vi "Dresden R2R Sputter 03.02.2018 IY24.vi"() -> ()   [LabVIEW 2009] (continued)
                                }
                                frame #1 {
                                n31817 = while {
                                i -> [w36487]
                                stop <- w36484 stop-if-true
                                n31818 = Greater?(x=w36487, y=50 ("Baratron set zero time 2")) -> (0:w36486:bool)
                                n31819 = case shown="True" w36486 {
                                frame #0 {
                                }
                                frame #1 {
                                n31820 = local write "Semi"(TRUE ("Semi")) -> ()
                                n31821 = local write "Error Message"("" ("Error Message")) -> ()
                                }
                                }
                                n31822 = local read "Pressure_ch3"() -> (w36483:i32)
                                n31823 = Less?(x=w36483, y=0.1 ("Pressure Check for baratron set zero")) -> (x < y?=w36490:bool)
                                n31824 = case shown="False" w36490 {
                                tunnel: [FALSE TRUE] -> w36489
                                frame #0 {
                                n31825 = Wait Until Next ms Multiple(millisecond multiple=u32 200) -> ()  [unwired: 1 out]
                                }
                                frame #1 {
                                }
                                }
                                n31826 = local read "Semi"() -> (w36488:bool)
                                n31827 = Or(x=w36489, y=w36488) -> (x .or. y?=w36484:bool)
                                }
                                }
                                frame #2 {
                                n31828 = local read "Semi"() -> (w36497:bool)
                                n31829 = case shown="False" w36497 {
                                frame #0 {
                                n31830 = local write "SDC1 2b"(TRUE ("SDC1 2b")) -> ()
                                n31831 = Wait (ms)(milliseconds to wait=u32 1000) -> ()  [unwired: 1 out]
                                }
                                frame #1 {
                                }
                                }
                                }
                                }
                                }
                                frame #3 {
                                # "CC CLOSE"
                                n31832 = stacked-sequence {
                                frame #0 {
                                n31833 = local read "Semi"() -> (w36500:bool)
                                n31834 = case shown="False" w36500 {
                                frame #0 {
                                n31835 = while {
                                i -> [w36506]
                                stop <- w36501 stop-if-true
                                n31836 = Greater?(x=w36506, y=50) -> (0:w36505:bool)
                                n31837 = case shown="True" w36505 {
                                frame #0 {
                                }
                                frame #1 {
                                n31838 = local write "Semi"(TRUE ("Semi")) -> ()
                                n31839 = local write "Error Message"("Coating Process  \nwas cancelled.\nPlease check \nBG-BV connection." ("Error Message")) -> ()
                                }
                                }
                                n31840 = local read "Ch3_Cc_on_off_di"() -> (w36504:bool)
                                n31841 = case shown="True" w36504 {
                                tunnel: [TRUE FALSE] -> w36503
                                frame #0 {
                                }
                                frame #1 {
                                n31842 = local write "Ch3_Cc_on_off_do"(FALSE ("Ch1_WFC_do")) -> ()
                                n31843 = Wait Until Next ms Multiple(millisecond multiple=u32 200) -> ()  [unwired: 1 out]
                                }
                                }
                                n31844 = local read "Semi"() -> (w36502:bool)
                                n31845 = Or(x=w36503, y=w36502) -> (x .or. y?=w36501:bool)
                                }
                                }
                                frame #1 {
                                }
                                }
                                }
                                frame #1 {
                                n31846 = local read "Semi"() -> (w36514:bool)
                                n31847 = case shown="False" w36514 {
                                frame #0 {
                                n31848 = local write "SDC1 3"(TRUE ("SDC1 3")) -> ()
                                n31849 = Wait (ms)(milliseconds to wait=u32 1000) -> ()  [unwired: 1 out]
                                }
                                frame #1 {
                                }
                                }
                                }
                                }
                                }
                                frame #4 {
                                # "PC-BV CLOSE"
                                n31850 = stacked-sequence {
                                frame #0 {
                                n31851 = local read "Semi"() -> (w36517:bool)
                                n31852 = case shown="False" w36517 {
                                frame #0 {
                                n31853 = stacked-sequence {
                                frame #0 {
                                n31854 = local read "Semi"() -> (w36518:bool)
                                n31855 = case shown="False" w36518 {
                                frame #0 {
                                n31856 = local write "Pc_bv3_auto_close"(TRUE ("Tp1_auto_start")) -> ()
                                }
                                frame #1 {
                                }
                                }
                                }
                                frame #1 {
                                n31857 = local read "Semi"() -> (w36520:bool)
                                n31858 = case shown="False" w36520 {
                                frame #0 {
                                n31859 = Wait (ms)(milliseconds to wait=u32 1000) -> ()  [unwired: 1 out]
                                }
                                frame #1 {
                                }
                                }
                                }
                                frame #2 {
                                n31860 = local read "Semi"() -> (w36522:bool)
                                n31861 = case shown="False" w36522 {
                                frame #0 {
                                n31862 = while {
                                i -> [w36528]
                                stop <- w36524 stop-if-true
                                n31863 = local read "Pc_bv_closed_ch3"() -> (w36526:bool)
                                n31864 = Greater?(x=w36528, y=120) -> (0:w36527:bool)
                                n31865 = local read "Semi"() -> (w36525:bool)
                                n31866 = Compound Arithmetic op=OR(w36525, w36526, w36527) -> (w36524:bool)
                                n31867 = Wait (ms)(milliseconds to wait=u32 500) -> ()  [unwired: 1 out]
                                }
                                }
                                frame #1 {
                                }
                                }
                                }
                                frame #3 {
                                n31868 = local read "Semi"() -> (w36530:bool)
                                n31869 = case shown="False" w36530 {
                                frame #0 {
                                n31870 = local read "Pc_bv_closed_ch3"() -> (w36531:bool)
                                n31871 = case shown="False" w36531 {
                                frame #0 {
                                n31872 = local write "Pc_bv3_auto_close"(TRUE ("Pc_bv1_auto_open")) -> ()
                                }
                                frame #1 {
                                }
                                }
                                }
                                frame #1 {
                                }
                                }
                                }
                                frame #4 {
                                n31873 = local read "Semi"() -> (w36533:bool)
                                n31874 = case shown="False" w36533 {
                                frame #0 {
                                n31875 = local read "Pc_bv_closed_ch3"() -> (w36534:bool)
                                n31876 = case shown="False" w36534 {
                                frame #0 {
                                n31877 = Wait (ms)(milliseconds to wait=u32 1000) -> ()  [unwired: 1 out]
                                }
                                frame #1 {
                                }
                                }
                                }
                                frame #1 {
                                }
                                }
                                }
                                frame #5 {
                                n31878 = local read "Semi"() -> (w36536:bool)
                                n31879 = case shown="False" w36536 {
                                frame #0 {
                                n31880 = while {
                                i -> [w36542]
                                stop <- w36538 stop-if-true
                                n31881 = local read "Pc_bv_closed_ch3"() -> (w36540:bool)
                                n31882 = Greater?(x=w36542, y=120) -> (0:w36541:bool)
                                n31883 = local read "Semi"() -> (w36539:bool)
                                n31884 = Compound Arithmetic op=OR(w36539, w36540, w36541) -> (w36538:bool)
                                n31885 = Wait (ms)(milliseconds to wait=u32 500) -> ()  [unwired: 1 out]
                                }
                                }
                                frame #1 {
                                }
                                }
                                }
                                frame #6 {
                                n31886 = local read "Semi"() -> (w36544:bool)
                                n31887 = case shown="False" w36544 {
                                frame #0 {
                                n31888 = local read "Pc_bv_closed_ch3"() -> (w36545:bool)
                                n31889 = case shown="False" w36545 {
                                frame #0 {
                                n31890 = local write "Error Message"("Start up process  cancelled\nbecause  PC-BV not closed.\nPlease check PC-BV1 connections." ("Error Message")) -> ()
                                n31891 = Wait (ms)(milliseconds to wait=u32 1000) -> ()  [unwired: 1 out]
                                }
                                frame #1 {
                                }
                                }
                                }
                                frame #1 {
                                }
                                }
                                }
                                }
                                }
                                frame #1 {
                                }
                                }
                                }
                                frame #1 {
                                n31892 = local read "Semi"() -> (w36548:bool)
                                n31893 = case shown="False" w36548 {
                                frame #0 {
                                n31894 = local write "SDC1 5"(TRUE ("SDC1 5")) -> ()
                                n31895 = Wait (ms)(milliseconds to wait=u32 1000) -> ()  [unwired: 1 out]
                                }
                                frame #1 {
                                }
                                }
                                }
                                }
                                }
                                frame #5 {
                                # "SOV-AR OPEN"
                                n31896 = stacked-sequence {
                                frame #0 {
                                n31897 = local read "Semi"() -> (w36551:bool)
                                n31898 = case shown="False" w36551 {
                                frame #0 {
                                n31899 = while {
                                i -> [w36557]
                                stop <- w36552 stop-if-true
                                n31900 = Greater?(x=w36557, y=50) -> (0:w36556:bool)
                                n31901 = case shown="True" w36556 {
                                frame #0 {
                                }
                                frame #1 {
                                n31902 = local write "Semi"(TRUE ("Semi")) -> ()
                                n31903 = local write "Error Message"("Coating Process  \nwas cancelled.\nPlease check \nSOV-Ar connection." ("Error Message")) -> ()
                                }
                                }
                                n31904 = local read "Ch3_Sov_Ar_di"() -> (w36555:bool)
                                n31905 = case shown="False" w36555 {
                                tunnel: [FALSE TRUE] -> w36554
                                frame #0 {
                                n31906 = local write "Ch3_Sov_Ar_do"(TRUE ("Ch1_WFC_do")) -> ()
                                n31907 = Wait Until Next ms Multiple(millisecond multiple=u32 200) -> ()  [unwired: 1 out]
                                }
                                frame #1 {
                                }
                                }
                                n31908 = local read "Semi"() -> (w36553:bool)
                                n31909 = Or(x=w36554, y=w36553) -> (x .or. y?=w36552:bool)
                                }
                                }
                                frame #1 {
                                }
                                }
                                }
                                frame #1 {
                                n31910 = local read "Semi"() -> (w36565:bool)
                                n31911 = case shown="False" w36565 {
                                frame #0 {
                                n31912 = while {
                                i -> [w36570]
                                stop <- w36568 stop-if-true
                                n31913 = Greater?(x=w36570, y=5) -> (0:w36566:bool)
                                n31914 = Wait Until Next ms Multiple(millisecond multiple=u32 1000) -> ()  [unwired: 1 out]
                                n31915 = local read "Semi"() -> (w36569:bool)
                                n31916 = Or(x=w36566, y=w36569) -> (x .or. y?=w36568:bool)
                                }
                                }
                                frame #1 {
                                }
                                }
                                }
                                frame #2 {
                                n31917 = local read "Semi"() -> (w36572:bool)
                                n31918 = case shown="False" w36572 {
                                frame #0 {
                                n31919 = local write "SDC1 6"(TRUE ("SDC1 6")) -> ()
                                n31920 = Wait (ms)(milliseconds to wait=u32 1000) -> ()  [unwired: 1 out]
                                }
                                frame #1 {
                                }
                                }
                                }
                                }
                                }
                                frame #6 {
                                # "CHECK CHAMBER PRESSURE"
                                n31921 = stacked-sequence {
                                frame #0 {
                                n31922 = local read "Semi"() -> (w36575:bool)
                                n31923 = case shown="False" w36575 {
                                frame #0 {
                                n31924 = while {
                                i -> [w36583]
                                stop <- w36577 stop-if-true
                                n31925 = Greater?(x=w36583, y=300) -> (0:w36582:bool)
                                n31926 = case shown="True" w36582 {
                                frame #0 {
                                }
                                frame #1 {
                                n31927 = local write "Semi"(TRUE ("Semi")) -> ()
                                n31928 = local write "Error Message"("Coating Process cancelled.\nPlease check chamber \nconnections." ("Error Message")) -> ()
                                }
                                }
                                n31929 = local read "Ch_pg_press_ch3_gui"() -> (w36576:dbl)
                                n31930 = Greater Or Equal?(x=w36576, y=0.9 ("CHAMBER PRESSURE 4")) -> (x >= y?=w36580:bool)
                                n31931 = case shown="True" w36580 {
                                tunnel: [TRUE FALSE] -> w36579
                                frame #0 {
                                }
                                frame #1 {
                                n31932 = Wait Until Next ms Multiple(millisecond multiple=u32 200) -> ()  [unwired: 1 out]
                                }
                                }
                                n31933 = local read "Semi"() -> (w36578:bool)
                                n31934 = Or(x=w36579, y=w36578) -> (x .or. y?=w36577:bool)
                                }
                                }
                                frame #1 {
                                }
                                }
                                }
                                frame #1 {
                                n31935 = local read "Semi"() -> (w36590:bool)
                                n31936 = case shown="False" w36590 {
                                frame #0 {
                                n31937 = Wait (ms)(milliseconds to wait=u32 1000) -> ()  [unwired: 1 out]
                                n31938 = local write "SDC1 8"(TRUE ("SDC1 8")) -> ()
                                }
                                frame #1 {
                                }
                                }
                                }
                                }
                                }
                                frame #7 {
                                # "PC-BV OPEN"
                                n31939 = stacked-sequence {
                                frame #0 {
                                n31940 = local read "Semi"() -> (w36593:bool)
                                n31941 = case shown="False" w36593 {
                                frame #0 {
                                n31942 = stacked-sequence {
                                frame #0 {
                                n31943 = local read "Semi"() -> (w36594:bool)
                                n31944 = case shown="False" w36594 {
                                frame #0 {
                                n31945 = local write "Pc_bv3_auto_open"(TRUE ("Tp1_auto_start")) -> ()
                                }
                                frame #1 {
                                }
                                }
                                }
                                frame #1 {
                                n31946 = local read "Semi"() -> (w36596:bool)
                                n31947 = case shown="False" w36596 {
                                frame #0 {
                                n31948 = Wait (ms)(milliseconds to wait=u32 1000) -> ()  [unwired: 1 out]
                                }
                                frame #1 {
                                }
                                }
                                }
                                frame #2 {
                                n31949 = local read "Semi"() -> (w36598:bool)
                                n31950 = case shown="False" w36598 {
                                frame #0 {
                                n31951 = while {
                                i -> [w36604]
                                stop <- w36600 stop-if-true
                                n31952 = local read "Pc_bv_opened_ch3"() -> (w36602:bool)
                                n31953 = Greater?(x=w36604, y=120) -> (0:w36603:bool)
                                n31954 = local read "Semi"() -> (w36601:bool)
                                n31955 = Compound Arithmetic op=OR(w36601, w36602, w36603) -> (w36600:bool)
                                n31956 = Wait (ms)(milliseconds to wait=u32 500) -> ()  [unwired: 1 out]
                                }
                                }
                                frame #1 {
                                }
                                }
                                }
                                frame #3 {
                                n31957 = local read "Semi"() -> (w36606:bool)
                                n31958 = case shown="False" w36606 {
                                frame #0 {
                                n31959 = local read "Pc_bv_opened_ch3"() -> (w36607:bool)
                                n31960 = case shown="False" w36607 {
                                frame #0 {
                                n31961 = local write "Pc_bv3_auto_open"(TRUE ("Pc_bv1_auto_open")) -> ()
                                }
                                frame #1 {
                                }
                                }
                                }
                                frame #1 {
                                }
                                }
                                }
                                frame #4 {
                                n31962 = local read "Semi"() -> (w36609:bool)
                                n31963 = case shown="False" w36609 {
                                frame #0 {
                                n31964 = local read "Pc_bv_opened_ch3"() -> (w36610:bool)
                                n31965 = case shown="False" w36610 {
                                frame #0 {
                                n31966 = Wait (ms)(milliseconds to wait=u32 1000) -> ()  [unwired: 1 out]
                                }
                                frame #1 {
                                }
                                }
                                }
                                frame #1 {
                                }
                                }
                                }
                                frame #5 {
                                n31967 = local read "Semi"() -> (w36612:bool)
                                n31968 = case shown="False" w36612 {
                                frame #0 {
                                n31969 = while {
                                i -> [w36618]
                                stop <- w36614 stop-if-true
                                n31970 = local read "Pc_bv_opened_ch3"() -> (w36616:bool)
                                n31971 = Greater?(x=w36618, y=120) -> (0:w36617:bool)
                                n31972 = local read "Semi"() -> (w36615:bool)
                                n31973 = Compound Arithmetic op=OR(w36615, w36616, w36617) -> (w36614:bool)
                                n31974 = Wait (ms)(milliseconds to wait=u32 500) -> ()  [unwired: 1 out]
                                }
                                }
                                frame #1 {
                                }
                                }
                                }
                                frame #6 {
                                n31975 = local read "Semi"() -> (w36620:bool)
                                n31976 = case shown="False" w36620 {
                                frame #0 {
                                n31977 = local read "Pc_bv_opened_ch3"() -> (w36621:bool)
                                n31978 = case shown="False" w36621 {
                                frame #0 {
                                n31979 = local write "Error Message"("Start up process  cancelled\nbecause  PC-BV not opened.\nPlease check PC-BV1 connections." ("Error Message")) -> ()
                                n31980 = Wait (ms)(milliseconds to wait=u32 1000) -> ()  [unwired: 1 out]
                                }
                                frame #1 {
                                }
                                }
                                }
                                frame #1 {
                                }
                                }
                                }
                                }
                                }
                                frame #1 {
                                }
                                }
                                }
                                frame #1 {
                                n31981 = local read "Semi"() -> (w36624:bool)
                                n31982 = case shown="False" w36624 {
                                frame #0 {
                                n31983 = Wait (ms)(milliseconds to wait=u32 1000) -> ()  [unwired: 1 out]
                                n31984 = local write "SDC1 7"(TRUE ("SDC1 7")) -> ()
                                }
                                frame #1 {
                                }
                                }
                                }
                                }
                                }
                                frame #8 {
                                # "CC OPEN"
                                n31985 = stacked-sequence {
                                frame #0 {
                                n31986 = local read "Semi"() -> (w36627:bool)
                                n31987 = case shown="False" w36627 {
                                frame #0 {
                                n31988 = while {
                                i -> [w36633]
                                stop <- w36628 stop-if-true
                                n31989 = Greater?(x=w36633, y=50) -> (0:w36632:bool)
                                n31990 = case shown="True" w36632 {
                                frame #0 {
                                }
                                frame #1 {
                                n31991 = local write "Semi"(TRUE ("Semi")) -> ()
                                n31992 = local write "Error Message"("Coating Process  \nwas cancelled.\nPlease check \nBG-BV connection." ("Error Message")) -> ()
                                }
                                }
                                n31993 = local read "Ch3_Cc_on_off_di"() -> (w36631:bool)
                                n31994 = case shown="False" w36631 {
                                tunnel: [FALSE TRUE] -> w36630
                                frame #0 {
                                n31995 = local write "Ch3_Cc_on_off_do"(TRUE ("Ch1_WFC_do")) -> ()
                                n31996 = Wait Until Next ms Multiple(millisecond multiple=u32 200) -> ()  [unwired: 1 out]
                                }
                                frame #1 {
                                }
                                }
                                n31997 = local read "Semi"() -> (w36629:bool)
                                n31998 = Or(x=w36630, y=w36629) -> (x .or. y?=w36628:bool)
                                }
                                }
                                frame #1 {
                                }
                                }
                                }
                                frame #1 {
                                n31999 = local read "Semi"() -> (w36641:bool)
                                n32000 = case shown="False" w36641 {
                                frame #0 {
                                n32001 = while {
                                i -> [w36646]
                                stop <- w36644 stop-if-true
                                n32002 = Greater?(x=w36646, y=30) -> (0:w36642:bool)
                                n32003 = Wait Until Next ms Multiple(millisecond multiple=u32 1000) -> ()  [unwired: 1 out]
                                n32004 = local read "Semi"() -> (w36645:bool)
                                n32005 = Or(x=w36642, y=w36645) -> (x .or. y?=w36644:bool)
                                }
                                }
                                frame #1 {
                                }
                                }
                                }
                                frame #2 {
                                n32006 = local read "Semi"() -> (w36648:bool)
                                n32007 = case shown="False" w36648 {
                                frame #0 {
                                n32008 = Wait (ms)(milliseconds to wait=u32 1000) -> ()  [unwired: 1 out]
                                n32009 = local write "SDC1 7b"(TRUE ("SDC1 3")) -> ()
                                }
                                frame #1 {
                                }
                                }
                                }
                                }
                                }
                                frame #9 {
                                # "CHECK CHAMBER PRESSURE"
                                n32010 = stacked-sequence {
                                frame #0 {
                                n32011 = local read "Semi"() -> (w36651:bool)
                                n32012 = case shown="False" w36651 {
                                frame #0 {
                                n32013 = while {
                                i -> [w36659]
                                stop <- w36653 stop-if-true
                                n32014 = Greater?(x=w36659, y=300) -> (0:w36658:bool)
                                n32015 = case shown="True" w36658 {
                                frame #0 {
                                }
                                frame #1 {
                                n32016 = local write "Semi"(TRUE ("Semi")) -> ()
                                n32017 = local write "Error Message"("Coating Process cancelled.\nPlease check chamber \nconnections." ("Error Message")) -> ()
                                }
                                }
                                n32018 = local read "Ch_CC_press_ch3 2"() -> (w36652:dbl)
                                n32019 = Greater Or Equal?(x=w36652, y=5e-05 ("CHAMBER PRESSURE 5")) -> (x >= y?=w36656:bool)
                                n32020 = case shown="True" w36656 {
                                tunnel: [TRUE FALSE] -> w36655
                                frame #0 {
                                }
                                frame #1 {
                                n32021 = Wait Until Next ms Multiple(millisecond multiple=u32 200) -> ()  [unwired: 1 out]
                                }
                                }
                                n32022 = local read "Semi"() -> (w36654:bool)
                                n32023 = Or(x=w36655, y=w36654) -> (x .or. y?=w36653:bool)
                                }
                                }
                                frame #1 {
                                }
                                }
                                }
                                frame #1 {
                                n32024 = local read "Semi"() -> (w36666:bool)
                                n32025 = case shown="False" w36666 {
                                frame #0 {
                                n32026 = Wait (ms)(milliseconds to wait=u32 1000) -> ()  [unwired: 1 out]
                                n32027 = local write "SDC1 10"(TRUE ("SDC1 10")) -> ()
                                }
                                frame #1 {
                                }
                                }
                                }
                                }
                                }
                                frame #10 {
                                # "CC CLOSE"
                                n32028 = stacked-sequence {
                                frame #0 {
                                n32029 = local read "Semi"() -> (w36669:bool)
                                n32030 = case shown="False" w36669 {
                                frame #0 {
                                n32031 = while {
                                i -> [w36675]
                                stop <- w36670 stop-if-true
                                n32032 = Greater?(x=w36675, y=50) -> (0:w36674:bool)
                                n32033 = case shown="True" w36674 {
                                frame #0 {
                                }
                                frame #1 {
                                n32034 = local write "Semi"(TRUE ("Semi")) -> ()
                                n32035 = local write "Error Message"("Coating Process  \nwas cancelled.\nPlease check \nBG-BV connection." ("Error Message")) -> ()
                                }
                                }
                                n32036 = local read "Ch3_Cc_on_off_di"() -> (w36673:bool)
                                n32037 = case shown="True" w36673 {
                                tunnel: [TRUE FALSE] -> w36672
                                frame #0 {
                                }
                                frame #1 {
                                n32038 = local write "Ch3_Cc_on_off_do"(FALSE ("Ch1_WFC_do")) -> ()
                                n32039 = Wait Until Next ms Multiple(millisecond multiple=u32 200) -> ()  [unwired: 1 out]
                                }
                                }
                                n32040 = local read "Semi"() -> (w36671:bool)
                                n32041 = Or(x=w36672, y=w36671) -> (x .or. y?=w36670:bool)
                                }
                                }
                                frame #1 {
                                }
                                }
                                }
                                frame #1 {
                                n32042 = local read "Semi"() -> (w36683:bool)
                                n32043 = case shown="False" w36683 {
                                frame #0 {
                                n32044 = local write "SDC1 10b"(TRUE ("SDC1 3")) -> ()
                                n32045 = Wait (ms)(milliseconds to wait=u32 1000) -> ()  [unwired: 1 out]
                                }
                                frame #1 {
                                }
                                }
                                }
                                }
                                }
                                frame #11 {
                                # "DC -Ignite Plasma"
                                n32046 = stacked-sequence {
                                frame #0 {
                                n32047 = local read "Semi"() -> (w36686:bool)
                                n32048 = case shown="False" w36686 {
                                frame #0 {
                                n32049 = stacked-sequence {
                                frame #0 {
                                n32050 = local read "Semi"() -> (w36687:bool)
                                n32051 = case shown="False" w36687 {
                                frame #0 {
                                n32052 = while {
                                i -> [w36693]
                                stop <- w36688 stop-if-true
                                n32053 = Greater?(x=w36693, y=50) -> (0:w36692:bool)
                                n32054 = case shown="True" w36692 {
                                frame #0 {
                                }
                                frame #1 {
                                n32055 = local write "Semi"(TRUE ("Semi")) -> ()
                                n32056 = local write "Error Message"("Sputtering Process cancelled.\nPlease check \nDC switch connections." ("Error Message")) -> ()
                                }
                                }
                                n32057 = local read "Cnt_Dcps_sw2_di"() -> (w36691:bool)
                                n32058 = case shown="False" w36691 {
                                tunnel: [FALSE ("Cnt_Dcps_sw1_do") TRUE ("Cnt_Dcps_sw1_do")] -> w36690
                                frame #0 {
                                n32059 = local write "Cnt_Dcps_sw2_do"(TRUE ("Cnt_Dcps_sw1_do")) -> ()
                                n32060 = Wait Until Next ms Multiple(millisecond multiple=u32 200) -> ()  [unwired: 1 out]
                                }
                                frame #1 {
                                }
                                }
                                n32061 = local read "Semi"() -> (w36689:bool)
                                n32062 = Or(x=w36690, y=w36689) -> (x .or. y?=w36688:bool)
                                }
                                }
                                frame #1 {
                                }
                                }
                                }
                                frame #1 {
                                n32063 = local read "Semi"() -> (w36701:bool)
                                n32064 = case shown="False" w36701 {
                                frame #0 {
                                n32065 = while {
                                i -> [w36707]
                                stop <- w36702 stop-if-true
                                n32066 = Greater?(x=w36707, y=50) -> (0:w36706:bool)
                                n32067 = case shown="True" w36706 {
                                frame #0 {
                                }
                                frame #1 {
                                n32068 = local write "Semi"(TRUE ("Semi")) -> ()
                                n32069 = local write "Error Message"("Sputtering Process cancelled.\nPlease check \nDC switch connections." ("Error Message")) -> ()
                                }
                                }
                                n32070 = local read "Cnt_Dcps_sw1_di"() -> (w36705:bool)
                                n32071 = case shown="True" w36705 {
                                tunnel: [TRUE ("Cnt_Dcps_sw1_do") FALSE ("Cnt_Dcps_sw1_do")] -> w36704
                                frame #0 {
                                }
                                frame #1 {
                                n32072 = local write "Cnt_Dcps_sw1_do"(FALSE ("Cnt_Dcps_sw1_do")) -> ()
                                n32073 = Wait Until Next ms Multiple(millisecond multiple=u32 200) -> ()  [unwired: 1 out]
                                }
                                }
                                n32074 = local read "Semi"() -> (w36703:bool)
                                n32075 = Or(x=w36704, y=w36703) -> (x .or. y?=w36702:bool)
                                }
                                }
                                frame #1 {
                                }
                                }
                                }
                                frame #2 {
                                n32076 = local read "Semi"() -> (w36715:bool)
                                n32077 = case shown="False" w36715 {
                                frame #0 {
                                n32078 = local write "Dc_host_auto"(TRUE ("Dc_host_auto")) -> ()
                                }
                                frame #1 {
                                }
                                }
                                }
                                frame #3 {
                                n32079 = local read "Semi"() -> (w36717:bool)
                                n32080 = case shown="False" w36717 {
                                frame #0 {
                                n32081 = local read "R Cmb Ch3 Step1 Coating Power"() -> (w36718:dbl)
                                n32082 = local write "Set DC Power       : 2"(w36718) -> ()
                                }
                                frame #1 {
                                }
                                }
                                }
                                frame #4 {
                                n32083 = local read "Semi"() -> (w36719:bool)
                                n32084 = case shown="False" w36719 {
                                frame #0 {
                                n32085 = Wait (ms)(milliseconds to wait=u32 1000) -> ()  [unwired: 1 out]
                                }
                                frame #1 {
                                }
                                }
                                }
                                frame #5 {
                                n32086 = local read "Semi"() -> (w36721:bool)
                                n32087 = case shown="False" w36721 {
                                frame #0 {
                                n32088 = local write "Dc_auto_set"(TRUE ("Dc_auto_set")) -> ()
                                }
                                frame #1 {
                                }
                                }
                                }
                                frame #6 {
                                n32089 = local read "Semi"() -> (w36723:bool)
                                n32090 = case shown="False" w36723 {
                                frame #0 {
                                n32091 = Wait (ms)(milliseconds to wait=u32 1000) -> ()  [unwired: 1 out]
                                }
                                frame #1 {
                                }
                                }
                                }
                                }
                                }
                                frame #1 {
                                }
                                }
                                }
                                frame #1 {
                                n32092 = local read "Semi"() -> (w36725:bool)
                                n32093 = case shown="False" w36725 {
                                frame #0 {
                                n32094 = Wait (ms)(milliseconds to wait=u32 1000) -> ()  [unwired: 1 out]
                                n32095 = local write "SDC1 13"(TRUE ("SDC1 13")) -> ()
                                }
                                frame #1 {
                                }
                                }
                                }
                                }
                                }
                                frame #12 {
                                n32096 = stacked-sequence {
                                frame #0 {
                                n32097 = local read "R Maximum diameter"() -> (w36729:dbl)
                                n32098 = local read "R Web speed(cm/min)"() -> (w36731:dbl)
                                n32099 = local read "R Minimum diameter"() -> (w36728:dbl)
                                n32100 = local read "R Web thicness"() -> (w36730:dbl)
                                n32101 = Wait (ms)(milliseconds to wait=u32 100) -> ()  [unwired: 1 out]
                                n32102 = local write "Initial Min Diameter"(w36728) -> ()
                                n32103 = local write "Max Diameter"(w36729) -> ()
                                n32104 = local write "Web Thickness"(w36730) -> ()
                                n32105 = local write "Web Speed"(w36731) -> ()
                                }
                                frame #1 {
                                n32106 = local read "R Cmb Ch2 Step1 Coating Power Active"() -> (w36746:bool)